vi "CRYO_MASTER_FULL_RUN3.vi"() -> ()   [LabVIEW 2017] (continued)
              }
              frame #1 {
                w484 = "_" ("string")
                n232 = local read "Cycle #"() -> (w482:u32)
                n233 = call "LV_UNIXTIME.vi"("current time"=w474) -> ("date/time string"=w485:string)  [unwired: 9 in, 1 out]
                n234 = Format Value(format string="%06d", value (0)=w482) -> (output string=w481:string)  [unwired: 1 in]
                n235 = Concatenate Strings(w472, w485, w484, w481, w484, "page5.png" ("string")) -> (w479:string)
                n236 = invoke class="TabCtl (strict)" method="Get Image"(error in=errorcluster {"status"=FALSE, "code"=0, "source"=""} ("error in (no error)")) -> (error out=w475:errorcluster, "image data"=w477:T23)  [unwired: 5 in, 4 out]
                n237 = Build Path(base path=w486, name or relative path=w479) -> (appended path=w478:path)
                n238 = call <vilib>:"Write PNG File.vi"("error in (no error)"=w475, "image data"=w477, "path to PNG file"=w478) -> ("error out"=w473:errorcluster)  [unwired: 7 in, 1 out]
              }
            }
            n239 = local write "error out (frontpanel screenshots)"(w466) -> ()
          }
          frame #5 {
            n240 = flat-sequence {
              tunnel: w490 -> [w493]
              tunnel: [w493] -> w489
              tunnel: w491 -> [w508]
              tunnel: w489 -> [w496]
              tunnel: [w495] -> w488
              tunnel: w487 -> [w494]
              frame #0 {
                n241 = property class="TabCtl (strict)"("Val(Sgnl)"=T1."DMMs" ("Value (Signaling)")) -> ()  [unwired: 2 in, 2 out]
              }
              frame #1 {
                w506 = "_" ("string")
                n242 = local read "Cycle #"() -> (w504:u32)
                n243 = call "LV_UNIXTIME.vi"("current time"=w496) -> ("date/time string"=w507:string)  [unwired: 9 in, 1 out]
                n244 = Format Value(format string="%06d", value (0)=w504) -> (output string=w503:string)  [unwired: 1 in]
                n245 = Concatenate Strings(w494, w507, w506, w503, w506, "page6.png" ("string")) -> (w501:string)
                n246 = invoke class="TabCtl (strict)" method="Get Image"(error in=errorcluster {"status"=FALSE, "code"=0, "source"=""} ("error in (no error)")) -> (error out=w497:errorcluster, "image data"=w499:T23)  [unwired: 5 in, 4 out]
                n247 = Build Path(base path=w508, name or relative path=w501) -> (appended path=w500:path)
                n248 = call <vilib>:"Write PNG File.vi"("error in (no error)"=w497, "image data"=w499, "path to PNG file"=w500) -> ("error out"=w495:errorcluster)  [unwired: 7 in, 1 out]
              }
            }
            n249 = local write "error out (frontpanel screenshots)"(w488) -> ()
          }
          frame #6 {
            n250 = flat-sequence {
              tunnel: w512 -> [w515]
              tunnel: [w515] -> w511
              tunnel: w513 -> [w530]
              tunnel: w511 -> [w518]
              tunnel: [w517] -> w510
              tunnel: w509 -> [w516]
              frame #0 {
                n251 = property class="TabCtl (strict)"("Val(Sgnl)"=T1."DIAGRAM" ("Value (Signaling)")) -> ()  [unwired: 2 in, 2 out]
              }
              frame #1 {
                w528 = "_" ("string")
                n252 = local read "Cycle #"() -> (w526:u32)
                n253 = Format Value(format string="%06d", value (0)=w526) -> (output string=w525:string)  [unwired: 1 in]
                n254 = call "LV_UNIXTIME.vi"("current time"=w518) -> ("date/time string"=w529:string)  [unwired: 9 in, 1 out]
                n255 = Concatenate Strings(w516, w529, w528, w525, w528, "page7.png" ("string")) -> (w523:string)
                n256 = invoke class="TabCtl (strict)" method="Get Image"(error in=errorcluster {"status"=FALSE, "code"=0, "source"=""} ("error in (no error)")) -> (error out=w519:errorcluster, "image data"=w521:T23)  [unwired: 5 in, 4 out]
                n257 = Build Path(base path=w530, name or relative path=w523) -> (appended path=w522:path)
                n258 = call <vilib>:"Write PNG File.vi"("error in (no error)"=w519, "image data"=w521, "path to PNG file"=w522) -> ("error out"=w517:errorcluster)  [unwired: 7 in, 1 out]
              }
            }
            n259 = local write "error out (frontpanel screenshots)"(w510) -> ()
          }
          frame #7 {
            n260 = flat-sequence {
              tunnel: w534 -> [w537]
              tunnel: [w537] -> w533
              tunnel: w535 -> [w552]
              tunnel: w533 -> [w540]
              tunnel: [w539] -> w532
              tunnel: w531 -> [w538]
              frame #0 {
                n261 = property class="TabCtl (strict)"("Val(Sgnl)"=T1."CHF" ("Value (Signaling)")) -> ()  [unwired: 2 in, 2 out]
              }
              frame #1 {
                w550 = "_" ("string")
                n262 = local read "Cycle #"() -> (w548:u32)
                n263 = Format Value(format string="%06d", value (0)=w548) -> (output string=w547:string)  [unwired: 1 in]
                n264 = call "LV_UNIXTIME.vi"("current time"=w540) -> ("date/time string"=w551:string)  [unwired: 9 in, 1 out]
                n265 = Concatenate Strings(w538, w551, w550, w547, w550, "page8.png" ("string")) -> (w545:string)
                n266 = invoke class="TabCtl (strict)" method="Get Image"(error in=errorcluster {"status"=FALSE, "code"=0, "source"=""} ("error in (no error)")) -> (error out=w541:errorcluster, "image data"=w543:T23)  [unwired: 5 in, 4 out]
                n267 = Build Path(base path=w552, name or relative path=w545) -> (appended path=w544:path)
                n268 = call <vilib>:"Write PNG File.vi"("error in (no error)"=w541, "image data"=w543, "path to PNG file"=w544) -> ("error out"=w539:errorcluster)  [unwired: 7 in, 1 out]
              }
            }
            n269 = local write "error out (frontpanel screenshots)"(w532) -> ()
          }
          frame #8 {
            n270 = flat-sequence {
              tunnel: w556 -> [w559]
              tunnel: [w559] -> w555
              tunnel: w557 -> [w574]
              tunnel: w555 -> [w562]
              tunnel: [w561] -> w554
              tunnel: w553 -> [w560]
              frame #0 {
                n271 = property class="TabCtl (strict)"("Val(Sgnl)"=T1."(Plc. hld.)" ("Value (Signaling)")) -> ()  [unwired: 2 in, 2 out]
              }
              frame #1 {
                w572 = "_" ("string")
                n272 = local read "Cycle #"() -> (w570:u32)
                n273 = Format Value(format string="%06d", value (0)=w570) -> (output string=w569:string)  [unwired: 1 in]
                n274 = call "LV_UNIXTIME.vi"("current time"=w562) -> ("date/time string"=w573:string)  [unwired: 9 in, 1 out]
                n275 = Concatenate Strings(w560, w573, w572, w569, w572, "page8.png" ("string")) -> (w567:string)
                n276 = invoke class="TabCtl (strict)" method="Get Image"(error in=errorcluster {"status"=FALSE, "code"=0, "source"=""} ("error in (no error)")) -> (error out=w563:errorcluster, "image data"=w565:T23)  [unwired: 5 in, 4 out]
                n277 = Build Path(base path=w574, name or relative path=w567) -> (appended path=w566:path)
                n278 = call <vilib>:"Write PNG File.vi"("error in (no error)"=w563, "image data"=w565, "path to PNG file"=w566) -> ("error out"=w561:errorcluster)  [unwired: 7 in, 1 out]
              }
            }
            n279 = local write "error out (frontpanel screenshots)"(w554) -> ()
          }
          frame #9 {
            n280 = local write "Frontpanel screenshots"(FALSE ("Frontpanel screenshots")) -> ()
          }
        }
        "error out (frontpanel screenshots)" <- w373
        n281 = property class="TabCtl (strict)"("Val(Sgnl)"=w371) -> ()  [unwired: 2 in, 2 out]
      }
      event "Stop Button": Value Change {
        n282 = event-data() -> ()  [unwired: 1 in, 3 out]
      }
    }
    n283 = Wait (ms)(milliseconds to wait=u32 123) -> ()  [unwired: 1 out]
  }
  n284 = while {
    stop <- w581 stop-if-true
    n285 = event shown="[5] \"Plot selecter LSI218(1)     1      2     3     4\", \"Plot selecter LSI218(2)     1      2     3     4\", \"Plot selecter (USB6210)     1      2     3     4\", \"Plot selecter LSI336       1      2     3     4\", \"Plot selecter (USB6218)     1      2     3     4\", \"Plot selecter (HP34401A)     1      2     3     4\": Value Change" {
      selector: _ -> [_ _ _ _ _ _ _ _ _ _ _]
      dyn-events: _ -> [_ _ _ _ _ _ _ _ _ _ _]
      timeout: _ -> [_ _ _ _ _ _ _ _ _ _ _]
      tunnel: [_ _ _ _ _ _ _ _ _ _ TRUE] -> w581
      tunnel: [errorcluster {"status"=FALSE, "code"=0, "source"=""} ("error out") w585 _ _ _ _ w721 w738 w755 w772 errorcluster {"status"=FALSE, "code"=0, "source"=""} ("error out")] -> w577
      event Timeout {
        n286 = event-data() -> ()  [unwired: 1 in, 3 out]
      }
      event "log/linear 1": Value Change {
        n287 = event-data() -> ()  [unwired: 1 in, 6 out]
        n288 = flat-sequence {
          tunnel: [w586] -> w585
          frame #0 {
            n289 = Boolean To (0,1)(Boolean="log/linear 1") -> (0, 1=w591:i16)
            n290 = control-ref of="Graph 1"() -> (w587:refnum<vi>)
            n291 = property class="XYGraph (strict)"(reference=w587, error in=errorcluster {"status"=FALSE, "code"=0, "source"=""} ("error in (no error)"), "YScale.Mapping Mode"=w591) -> (error out=w589:errorcluster)  [unwired: 1 out]
            n292 = control-ref of="error out (USB6210)"() -> (w590:refnum<vi>)
            n293 = property class="Clust (strict)"(reference=w590, "Val(Sgnl)"=w589) -> (error out=w586:errorcluster)  [unwired: 1 in, 1 out]
          }
        }
      }
      event "log/linear 2": Value Change {
        n294 = event-data() -> ()  [unwired: 1 in, 6 out]
        n295 = flat-sequence {
          frame #0 {
            n296 = Boolean To (0,1)(Boolean="log/linear 2") -> (0, 1=w597:i16)
            n297 = control-ref of="Graph 2"() -> (w595:refnum<vi>)
            n298 = property class="XYGraph (strict)"(reference=w595, error in=errorcluster {"status"=FALSE, "code"=0, "source"=""} ("error in (no error)"), "YScale.Mapping Mode"=w597) -> (error out=w596:errorcluster)  [unwired: 1 out]
            n299 = control-ref of="error out (USB6210)"() -> (w594:refnum<vi>)
            n300 = property class="Clust (strict)"(reference=w594, "Value"=w596) -> ()  [unwired: 1 in, 2 out]
          }
        }
      }
      event "log/linear 3": Value Change {
        n301 = event-data() -> ()  [unwired: 1 in, 6 out]
        n302 = flat-sequence {
          frame #0 {
            n303 = Boolean To (0,1)(Boolean="log/linear 3") -> (0, 1=w603:i16)
            n304 = control-ref of="Graph 3"() -> (w599:refnum<vi>)
            n305 = property class="XYGraph (strict)"(reference=w599, error in=errorcluster {"status"=FALSE, "code"=0, "source"=""} ("error in (no error)"), "YScale.Mapping Mode"=w603) -> (error out=w602:errorcluster)  [unwired: 1 out]
            n306 = control-ref of="error out (USB6210)"() -> (w601:refnum<vi>)
            n307 = property class="Clust (strict)"(reference=w601, "Value"=w602) -> ()  [unwired: 1 in, 2 out]
          }
        }
      }
      event "log/linear 4": Value Change {
        n308 = event-data() -> ()  [unwired: 1 in, 6 out]
        n309 = flat-sequence {
          frame #0 {
            n310 = Boolean To (0,1)(Boolean="log/linear 4") -> (0, 1=w609:i16)
            n311 = control-ref of="Graph 4"() -> (w605:refnum<vi>)
            n312 = property class="XYGraph (strict)"(reference=w605, error in=errorcluster {"status"=FALSE, "code"=0, "source"=""} ("error in (no error)"), "YScale.Mapping Mode"=w609) -> (error out=w608:errorcluster)  [unwired: 1 out]
            n313 = control-ref of="error out (USB6210)"() -> (w607:refnum<vi>)
            n314 = property class="Clust (strict)"(reference=w607, "Value"=w608) -> ()  [unwired: 1 in, 2 out]
          }
        }
      }
      event "Plot selecter LSI218(1)\n    1      2     3     4", "Plot selecter LSI218(2)\n    1      2     3     4", "Plot selecter (USB6210)\n    1      2     3     4", "Plot selecter LSI336 \n     1      2     3     4", "Plot selecter (USB6218)\n    1      2     3     4", "Plot selecter (HP34401A)\n    1      2     3     4": Value Change {
        n315 = event-data() -> ()  [unwired: 1 in, 6 out]
        n316 = local read "Labels (HP34401 LM)"() -> (w616:string[])
        n317 = call "BuildPlotLegends.vi"("Plot selecter \n    1      2     3     4"="Plot selecter (HP34401A)\n    1      2     3     4", "AllLabels"=w616) -> ("Series 4"=w611:string[], "Series 3"=w612:string[], "Series 2"=w613:string[], "Series 1"=w614:string[])  [unwired: 6 in]
        n318 = local read "All Labels (USB6210)"() -> (w633:string[])
        n319 = local read "All Labels (USB6218)"() -> (w622:string[])
        n320 = local read "Labels LSI218 (1)"() -> (w635:string[])
        n321 = local read "Labels LSI218 (2)"() -> (w636:string[])
        n322 = local read "Labels LSI336"() -> (w628:string[])
        n323 = call "BuildPlotLegends_LSI218.vi"("Plot selecter (2)\n    1      2     3     5"="Plot selecter LSI218(2)\n    1      2     3     4", "Plot selecter (1)\n    1      2     3     4"="Plot selecter LSI218(1)\n    1      2     3     4", "Labels (2)"=w636, "Labels (1)"=w635) -> ("Series 4"=w646:string[], "Series 3"=w644:string[], "Series 2"=w642:string[], "Series 1"=w640:string[])  [unwired: 4 in]
        n324 = call "BuildPlotLegends.vi"("Plot selecter \n    1      2     3     4"="Plot selecter (USB6210)\n    1      2     3     4", "AllLabels"=w633) -> ("Series 4"=w645:string[], "Series 3"=w643:string[], "Series 2"=w641:string[], "Series 1"=w639:string[])  [unwired: 6 in]
        n325 = call "BuildPlotLegends.vi"("Plot selecter \n    1      2     3     4"="Plot selecter LSI336 \n     1      2     3     4", "AllLabels"=w628) -> ("Series 4"=w623:string[], "Series 3"=w624:string[], "Series 2"=w625:string[], "Series 1"=w626:string[])  [unwired: 6 in]
        n326 = call "BuildPlotLegends.vi"("Plot selecter \n    1      2     3     4"="Plot selecter (USB6218)\n    1      2     3     4", "AllLabels"=w622) -> ("Series 4"=w618:string[], "Series 3"=w617:string[], "Series 2"=w619:string[], "Series 1"=w620:string[])  [unwired: 6 in]
        n327 = Build Array (concatenate)(w641, w642, w625, w619, w613) -> (w630:string[])
        "Series 2" <- w630
        n328 = Build Array (concatenate)(w643, w644, w624, w617, w612) -> (w631:string[])
        "Series 3" <- w631
        n329 = Build Array (concatenate)(w645, w646, w623, w618, w611) -> (w632:string[])
        "Series 4" <- w632
        n330 = Build Array (concatenate)(w639, w640, w626, w620, w614) -> (w629:string[])
        "Series 1" <- w629
        n331 = stacked-sequence {
          tunnel: [w656 _ _ _] -> w650
          tunnel: [_ w674 _ _] -> w651
          tunnel: [_ _ w691 _] -> w649
          tunnel: [_ _ _ w708] -> w648
          tunnel: w629 -> [w654 _ _ _]
          tunnel: w630 -> [_ w672 _ _]
          tunnel: w631 -> [_ _ w689 _]
          tunnel: w632 -> [_ _ _ w706]
          frame #0 {
            n332 = Array Size(array=w654) -> (size(s)=w658:i32)
            n333 = control-ref of="Graph 1"() -> (w652:refnum<vi>)
            n334 = property class="XYGraph (strict)"(reference=w652) -> ("LegNumRows"=w653:u32)  [unwired: 1 in, 2 out]
            n335 = for {
              N: w653 -> [_]
              tunnel: w652 -> [w667]
              shift-right: [w665] -> w657
              shift-left: errorcluster {"status"=FALSE, "code"=0, "source"=""} ("error in (no error)") -> [w666]
              i -> [w669]
              n336 = property class="XYGraph (strict)"(reference=w667, error in=w666, "Active Plot"=w669, "Plot.Plot Name"="") -> (error out=w665:errorcluster)  [unwired: 1 out]
            }
            n337 = for {
              N: w658 -> [_]
              tunnel: w652 -> [w663]
              shift-right: [w661] -> w656
              shift-left: w657 -> [w662]
              tunnel: w654 -> [w660] mode=indexing
              i -> [w664]
              n338 = property class="XYGraph (strict)"(reference=w663, error in=w662, "Active Plot"=w664, "Plot.Plot Name"=w660, "Plot.Visible?"=TRUE ("Plot.Visible")) -> (error out=w661:errorcluster)  [unwired: 1 out]
            }
          }
          frame #1 {
            n339 = Array Size(array=w672) -> (size(s)=w676:i32)
            n340 = control-ref of="Graph 2"() -> (w671:refnum<vi>)
            n341 = property class="XYGraph (strict)"(reference=w671) -> ("LegNumRows"=w670:u32)  [unwired: 1 in, 2 out]
            n342 = for {
              N: w670 -> [_]
              shift-right: [w683] -> w675
              shift-left: errorcluster {"status"=FALSE, "code"=0, "source"=""} ("error in (no error)") -> [w684]
              tunnel: w671 -> [w682]
              i -> [w686]
              n343 = property class="XYGraph (strict)"(reference=w682, error in=w684, "Active Plot"=w686, "Plot.Plot Name"="") -> (error out=w683:errorcluster)  [unwired: 1 out]
            }
            n344 = for {
              N: w676 -> [_]
              shift-right: [w679] -> w674
              shift-left: w675 -> [w680]
              tunnel: w672 -> [w678] mode=indexing
              tunnel: w671 -> [w677]
              i -> [w681]
              n345 = property class="XYGraph (strict)"(reference=w677, error in=w680, "Active Plot"=w681, "Plot.Plot Name"=w678) -> (error out=w679:errorcluster)  [unwired: 1 out]
            }
          }
          frame #2 {
            n346 = Array Size(array=w689) -> (size(s)=w693:i32)
            n347 = control-ref of="Graph 3"() -> (w687:refnum<vi>)
            n348 = property class="XYGraph (strict)"(reference=w687) -> ("LegNumRows"=w688:u32)  [unwired: 1 in, 2 out]
            n349 = for {
              N: w688 -> [_]
              tunnel: w687 -> [w701]
              shift-right: [w699] -> w692
              shift-left: errorcluster {"status"=FALSE, "code"=0, "source"=""} ("error in (no error)") -> [w700]
              i -> [w703]
              n350 = property class="XYGraph (strict)"(reference=w701, error in=w700, "Active Plot"=w703, "Plot.Plot Name"="") -> (error out=w699:errorcluster)  [unwired: 1 out]
            }
            n351 = for {
              N: w693 -> [_]
              tunnel: w687 -> [w697]
              shift-right: [w695] -> w691
              shift-left: w692 -> [w696]
              tunnel: w689 -> [w694] mode=indexing
              i -> [w698]
              n352 = property class="XYGraph (strict)"(reference=w697, error in=w696, "Active Plot"=w698, "Plot.Plot Name"=w694) -> (error out=w695:errorcluster)  [unwired: 1 out]
            }
          }
          frame #3 {
            n353 = Array Size(array=w706) -> (size(s)=w710:i32)
            n354 = control-ref of="Graph 4"() -> (w704:refnum<vi>)
            n355 = property class="XYGraph (strict)"(reference=w704) -> ("LegNumRows"=w705:u32)  [unwired: 1 in, 2 out]
            n356 = for {
              N: w705 -> [_]
              tunnel: w704 -> [w718]
              shift-right: [w716] -> w709
              shift-left: errorcluster {"status"=FALSE, "code"=0, "source"=""} ("error in (no error)") -> [w717]
              i -> [w720]
              n357 = property class="XYGraph (strict)"(reference=w718, error in=w717, "Active Plot"=w720, "Plot.Plot Name"="") -> (error out=w716:errorcluster)  [unwired: 1 out]
            }
            n358 = for {
              N: w710 -> [_]
              tunnel: w704 -> [w714]
              shift-right: [w712] -> w708
              shift-left: w709 -> [w713]
              tunnel: w706 -> [w711] mode=indexing
              i -> [w715]
              n359 = property class="XYGraph (strict)"(reference=w714, error in=w713, "Active Plot"=w715, "Plot.Plot Name"=w711) -> (error out=w712:errorcluster)  [unwired: 1 out]
            }
          }
        }
        n360 = Merge Errors(w650, w651, w649, w648) -> (→"Plot errors":errorcluster)
      }
      event "Take Screenshot! 1": Value Change {
        n361 = event-data() -> ()  [unwired: 1 in, 6 out]
        n362 = flat-sequence {
          tunnel: [w722] -> w721
          frame #0 {
            n363 = flat-sequence {
              tunnel: [w723] -> w722
              frame #0 {
                w732 = "_" ("string")
                n364 = Get Date/Time In Seconds() -> (seconds since 1Jan1904=w729:timestamp)
                n365 = local read "RUN Identifier"() -> (w734:string)
                n366 = call "LV_UNIXTIME.vi"("current time"=w729) -> ("date/time string"=w733:string)  [unwired: 9 in, 1 out]
                n367 = control-ref of="Graph 1"() -> (w728:refnum<vi>)
                n368 = Concatenate Strings(w734, w732, w733, w732, "FIle suffix 1", ".png" ("string")) -> (w736:string)
                n369 = local read "Base Path"() -> (w735:path)
                n370 = invoke class="XYGraph (strict)" method="Get Image"(reference=w728, error in=errorcluster {"status"=FALSE, "code"=0, "source"=""} ("error in (no error)")) -> (error out=w724:errorcluster, "image data"=w727:T23)  [unwired: 4 in, 4 out]
                n371 = Build Path(base path=w735, name or relative path=w736) -> (appended path=w726:path)
                n372 = call <vilib>:"Write PNG File.vi"("error in (no error)"=w724, "image data"=w727, "path to PNG file"=w726) -> ("error out"=w723:errorcluster)  [unwired: 7 in, 1 out]
              }
              frame #1 {
                n373 = local write "Take Screenshot! 1"(FALSE ("Take Screenshot! 1")) -> ()
              }
            }
          }
        }
      }
      event "Take Screenshot! 2": Value Change {
        n374 = event-data() -> ()  [unwired: 1 in, 6 out]
        n375 = flat-sequence {
          tunnel: [w739] -> w738
          frame #0 {
            n376 = flat-sequence {
              tunnel: [w745] -> w739
              frame #0 {
                w749 = "_" ("string")
                n377 = Get Date/Time In Seconds() -> (seconds since 1Jan1904=w746:timestamp)
                n378 = local read "RUN Identifier"() -> (w751:string)
                n379 = call "LV_UNIXTIME.vi"("current time"=w746) -> ("date/time string"=w750:string)  [unwired: 9 in, 1 out]
                n380 = control-ref of="Graph 2"() -> (w740:refnum<vi>)
                n381 = Concatenate Strings(w751, w749, w750, w749, "FIle suffix 2", ".png" ("string")) -> (w753:string)
                n382 = local read "Base Path"() -> (w752:path)
                n383 = invoke class="XYGraph (strict)" method="Get Image"(reference=w740, error in=errorcluster {"status"=FALSE, "code"=0, "source"=""} ("error in (no error)")) -> (error out=w744:errorcluster, "image data"=w742:T23)  [unwired: 4 in, 4 out]
                n384 = Build Path(base path=w752, name or relative path=w753) -> (appended path=w741:path)
                n385 = call <vilib>:"Write PNG File.vi"("error in (no error)"=w744, "image data"=w742, "path to PNG file"=w741) -> ("error out"=w745:errorcluster)  [unwired: 7 in, 1 out]
              }
              frame #1 {
                n386 = local write "Take Screenshot! 2"(FALSE ("Take Screenshot! 1")) -> ()
              }
            }
          }
        }
      }
      event "Take Screenshot! 3": Value Change {
        n387 = event-data() -> ()  [unwired: 1 in, 6 out]
        n388 = flat-sequence {
          tunnel: [w756] -> w755
          frame #0 {
            n389 = flat-sequence {
              tunnel: [w758] -> w756
              frame #0 {
                w766 = "_" ("string")
                n390 = Get Date/Time In Seconds() -> (seconds since 1Jan1904=w764:timestamp)
                n391 = local read "RUN Identifier"() -> (w768:string)
                n392 = call "LV_UNIXTIME.vi"("current time"=w764) -> ("date/time string"=w767:string)  [unwired: 9 in, 1 out]
                n393 = control-ref of="Graph 3"() -> (w761:refnum<vi>)
                n394 = Concatenate Strings(w768, w766, w767, w766, "FIle suffix 3", ".png" ("string")) -> (w770:string)
                n395 = local read "Base Path"() -> (w769:path)
                n396 = invoke class="XYGraph (strict)" method="Get Image"(reference=w761, error in=errorcluster {"status"=FALSE, "code"=0, "source"=""} ("error in (no error)")) -> (error out=w759:errorcluster, "image data"=w757:T23)  [unwired: 4 in, 4 out]
                n397 = Build Path(base path=w769, name or relative path=w770) -> (appended path=w762:path)
                n398 = call <vilib>:"Write PNG File.vi"("error in (no error)"=w759, "image data"=w757, "path to PNG file"=w762) -> ("error out"=w758:errorcluster)  [unwired: 7 in, 1 out]
              }
              frame #1 {
                n399 = local write "Take Screenshot! 3"(FALSE ("Take Screenshot! 1")) -> ()
              }
            }
          }
        }
      }
      event "Take Screenshot! 4": Value Change {
        n400 = event-data() -> ()  [unwired: 1 in, 6 out]
        n401 = flat-sequence {
          tunnel: [w773] -> w772
          frame #0 {
            n402 = flat-sequence {
              tunnel: [w776] -> w773
              frame #0 {
                w783 = "_" ("string")
                n403 = Get Date/Time In Seconds() -> (seconds since 1Jan1904=w781:timestamp)
                n404 = local read "RUN Identifier"() -> (w785:string)
                n405 = call "LV_UNIXTIME.vi"("current time"=w781) -> ("date/time string"=w784:string)  [unwired: 9 in, 1 out]
                n406 = control-ref of="Graph 4"() -> (w777:refnum<vi>)
                n407 = Concatenate Strings(w785, w783, w784, w783, "FIle suffix 4", ".png" ("string")) -> (w787:string)
                n408 = local read "Base Path"() -> (w786:path)
                n409 = invoke class="XYGraph (strict)" method="Get Image"(reference=w777, error in=errorcluster {"status"=FALSE, "code"=0, "source"=""} ("error in (no error)")) -> (error out=w774:errorcluster, "image data"=w778:T23)  [unwired: 4 in, 4 out]
                n410 = Build Path(base path=w786, name or relative path=w787) -> (appended path=w779:path)
                n411 = call <vilib>:"Write PNG File.vi"("error in (no error)"=w774, "image data"=w778, "path to PNG file"=w779) -> ("error out"=w776:errorcluster)  [unwired: 7 in, 1 out]
              }
              frame #1 {
                n412 = local write "Take Screenshot! 4"(FALSE ("Take Screenshot! 1")) -> ()
              }
            }
          }
        }
      }
      event "Stop Button": Value Change {
        n413 = event-data() -> ()  [unwired: 1 in, 6 out]
      }
    }
    "error out (graph operations)" <- w577
    n414 = local write "Take Screenshot! 1"(FALSE ("Take Screenshot! 1")) -> ()
    n415 = local write "Take Screenshot! 2"(FALSE ("Take Screenshot! 1")) -> ()
    n416 = Wait (ms)(milliseconds to wait=u32 1000) -> ()  [unwired: 1 out]
    n417 = local write "Take Screenshot! 3"(FALSE ("Take Screenshot! 1")) -> ()
    n418 = local write "Take Screenshot! 4"(FALSE ("Take Screenshot! 1")) -> ()
  }
  n419 = while {
    i -> [w795]
    stop <- w792 stop-if-true
    n420 = Equal?(x=w795, y=0) -> (x = y?=w793:bool)
    n421 = case shown="True" w793 {
      frame False {
      }
      frame True {
        n422 = property on="Agilent\nIntialized?" class="Bool (strict)"("Val(Sgnl)"=FALSE ("Value (Signaling)")) -> ()  [unwired: 2 in, 2 out]
      }
    }
    n423 = Wait (ms)(milliseconds to wait=u32 123) -> ()  [unwired: 1 out]
    n424 = event shown="[4] \"V_lim_up (V)\", \"V_lim_low (V)\": Value Change" {
      selector: _ -> [_ _ _ _ _]
      dyn-events: _ -> [_ _ _ _ _]
      timeout: _ -> [_ _ _ _ _]
      tunnel: [FALSE ("Value (Signaling)") TRUE ("Value (Signaling)") _ _ _] -> w792
      tunnel: "VISA (Agilent 34402)" -> [_ _ w801 w804 _]
      event Timeout {
        n425 = event-data() -> ()  [unwired: 1 in, 3 out]
      }
      event "Stop Button": Value Change {
        n426 = event-data() -> ()  [unwired: 1 in, 3 out]
      }
      event "Initialize (Agilent)": Value Change {
        n427 = event-data() -> ()  [unwired: 1 in, 3 out]
        n428 = property on="Agilent\nIntialized?" class="Bool (strict)"("Val(Sgnl)"=TRUE ("Value (Signaling)")) -> ()  [unwired: 2 in, 2 out]
        n429 = call "Initialize.vi"("error in (no error)"=errorcluster {"status"=FALSE, "code"=0, "source"=""}, "VISA resource name"=w801) -> ("error out"=→"error out (Agilent)":errorcluster)  [unwired: 8 in, 1 out]
      }
      event "OUTPUT \nKenwood", "Kenwood set V (V)": Value Change {
        n430 = local read "Agilent\nIntialized?"() -> (w803:bool)
        n431 = event-data() -> ()  [unwired: 1 in, 3 out]
        n432 = case shown="True" w803 {
          tunnel: w804 -> [_ w810]
          frame False {
          }
          frame True {
            w812 = u16 0 items=["DC", "Sine", "Square", "Triangle", "Ramp", "Pulse", "Noise", "Sinc", "Negative Ramp", "Exponential Rise", "Exponential Fall", "Cardiac"] ("Waveform Function (1: Sine)")
            n433 = xnode "Formula"("X1"="Kenwood set V (V)") -> ("Result"=w805:dbl)  [unwired: 1 in, 1 out]
            n434 = call "Configure Standard Waveform.vi"("DC Offset (0.00 V)"=w805, "Frequency (1000 Hz)"=1.0, "error in (no error)"=errorcluster {"status"=FALSE, "code"=0, "source"=""}, "Amplitude (1)"=1.0, "Waveform Function (1: Sine)"=w812, "VISA resource name"=w810) -> ("error out"=w814:errorcluster, "VISA resource name out"=w815:refnum<visa-resource-name>)  [unwired: 4 in]
            n435 = call "Enable Output.vi"("error in (no error)"=w814, "Enable Output  (T: Enable)"="OUTPUT \nKenwood", "VISA resource name"=w815) -> ("error out"=w808:errorcluster)  [unwired: 7 in, 1 out]
            n436 = local write "error out (Agilent)"(w808) -> ()
          }
        }
      }
      event "V_lim_up (V)", "V_lim_low (V)": Value Change {
        n437 = event-data() -> ()  [unwired: 1 in, 3 out]
        n438 = property on="Kenwood set V (V)" class="DigNum (strict)"("Minimum"="V_lim_low (V)", "Maximum"="V_lim_up (V)") -> ()  [unwired: 2 in, 2 out]
      }
    }
  }
  n439 = while {
    stop <- w827 stop-if-true
    n440 = Wait (ms)(milliseconds to wait=u32 101) -> ()  [unwired: 1 out]
    n441 = event shown="[2] Timeout" {
      selector: _ -> [_ _ _]
      dyn-events: _ -> [_ _ _]
      timeout: _ -> [_ _ _]
      tunnel: [FALSE TRUE FALSE] -> w827
      event "Initialize (DMMs)": Value Change {
        w830 = T4 [] ("Value (Signaling)")
        n442 = event-data() -> ()  [unwired: 1 in, 3 out]
        n443 = property on="Graph DMMs 1" class="XYGraph (strict)"("Val(Sgnl)"=w830) -> ()  [unwired: 2 in, 2 out]
        n444 = property on="Graph DMMs 2" class="XYGraph (strict)"("Val(Sgnl)"=w830) -> ()  [unwired: 2 in, 2 out]
      }
      event "Stop Button": Value Change {
        n445 = event-data() -> ()  [unwired: 1 in, 3 out]
      }
      event Timeout {
        n446 = event-data() -> ()  [unwired: 1 in, 3 out]
      }
    }
  }
  n447 = Obtain Notifier(name (unnamed)="stop notifier", notification data type=w17, create if not found? (T)=w17, error in (no error)=errorcluster {"status"=FALSE, "code"=0, "source"=""}) -> (notifier out=w5:refnum<notifier>, error out=w4:errorcluster)  [unwired: 1 out]
  n448 = while {
    shift-right: [w943] -> w40
    shift-left: refnum<class "USBData.lvclass"> refnum ("USBData.lvclass") -> [w946]
    shift-right: [w939] -> w39
    shift-left: w6 -> [w945]
    tunnel: "Base Path" -> [w845]
    shift-right: [w921] -> w34
    shift-left: errorcluster {"status"=FALSE, "code"=0, "source"=""} ("error in (no error)") -> [w937]
    shift-right: [w922] -> w35
    shift-left: refnum<class "LSI218Data.lvclass"> refnum ("LSI218Data.lvclass") -> [w936]
    shift-right: [w909] -> w31
    shift-left: refnum<class "LSI336Data.lvclass"> refnum ("LSI336Data.lvclass") -> [w918]
    shift-right: [w908] -> w30
    shift-left: w21 -> [w917]
    shift-right: [w897] -> _
    shift-left: w6 -> [w898]
    shift-right: [w887] -> w25
    shift-left: refnum<class "USBData.lvclass"> refnum ("USBData.lvclass") -> [w895]
    shift-right: [w886] -> w24
    shift-left: errorcluster {"status"=FALSE, "code"=0, "source"=""} ("error in (no error)") -> [w894]
    shift-right: [w883] -> _
    shift-left: w21 -> [w882]
    tunnel: w5 -> [w853]
    tunnel: w4 -> [w852]
    tunnel: [w850] -> w13
    tunnel: [w849] -> w12
    shift-right: [w846] -> _
    shift-left: refnum<class "LMData.lvclass"> refnum ("LMData in") -> [w847]
    shift-right: [w843] -> _
    shift-left: errorcluster {"status"=FALSE, "code"=0, "source"=""} ("error in (no error)") -> [w844]
    i -> [w842]
    stop <- "Stop Button" stop-if-true
    w838 = T25 [] ("appended array")
    w904 = u32 24 ("Number of Rows")
    w914 = T25 [] ("appended array")
    w931 = T25 [] ("appended array")
    n449 = local read "LSI218Settings(A-F)"() -> (w874:T3)
    n450 = control-ref of="Plot selecter LSI218(2)\n    1      2     3     4"() -> (w902:refnum<vi>)
    n451 = control-ref of="Plot selecter LSI218(1)\n    1      2     3     4"() -> (w903:refnum<vi>)
    n452 = control-ref of="Plot selecter LSI336 \n     1      2     3     4"() -> (w901:refnum<vi>)
    n453 = property on="Property Node" class="Arr (strict)"(reference=w902, "Number of Rows"=w904) -> ()  [unwired: 1 in, 2 out]
    n454 = property on="Property Node" class="Arr (strict)"(reference=w903, "Number of Rows"=w904) -> ()  [unwired: 1 in, 2 out]
    n455 = local read "LSI336Settings(X,Y)"() -> (w872:T3)
    n456 = Array Size(array=w874) -> (size(s)=w873:i32)
    n457 = property on="Property Node" class="Arr (strict)"(reference=w901, "Number of Rows"=u32 8) -> ()  [unwired: 1 in, 2 out]
    n458 = Multiply(x="Measurement Interval (s)", y=u32 1000) -> (x*y=w940:dbl)
    n459 = Wait (ms)(milliseconds to wait=w940) -> ()  [unwired: 1 out]
    n460 = for {
      N: w873 -> [_]
      tunnel: w874 -> [w1034] mode=indexing
      tunnel: [w1033] -> w870 mode=concatenating
      n461 = Unbundle By Name(w1034) -> ("SensorLocations"=w1033:T18)
    }
    n462 = for {
      tunnel: w872 -> [w1032] mode=indexing
      tunnel: [w1031] -> w871 mode=concatenating
      n463 = Unbundle By Name(w1032) -> ("SensorLocations"=w1031:T18)
    }
    n464 = Quotient & Remainder(x=w842, y="Screenshots interval") -> (x-y*floor(x/y)=w858:i64)  [unwired: 1 out]
    n465 = Equal?(x=w842, y=0) -> (x = y?=w848:bool)
    n466 = case shown="True" w848 {
      tunnel: w946 -> [w2099 w2122]
      tunnel: w945 -> [w2093 w2120]
      tunnel: w842 -> [w2084 _]
      tunnel: [w2091 w2117] -> w939
      tunnel: [w2088 w2116] -> w896
      tunnel: [w2089 w2115] -> w943
      tunnel: [w2079 w2110] -> w944
      tunnel: w845 -> [_ w2109]
      tunnel: [w2078 w2106] -> w879
      frame False {
        n467 = call-dynamic "USBData_measure.vi"("USBData in"=w2099, "DAQ sample #"=i64 5, "DAQ timeout"=100.0 ("DAQ timeout (def: 100)"), "MeasurementIndex"=w2084, "error in (no error)"=w2093, "save every ... measurements"="Record interval") -> ("USBData out"=w2098:refnum<class "USBData.lvclass">, "TimeMeasuremeent"=w2095:timestamp, "Status"=→"USB6210 Status":T6, "LastDataAcquired"=w2080:dbl[], "error out"=w2094:errorcluster)  [unwired: 3 in, 2 out]
        "Time of Last Measurement (USB6210)" <- w2095
        "Last Vol\n(USB6210)" <- w2080
        n468 = call-dynamic "USBData_convert.vi"("Save every ... measurements"="Record interval", "MeasurementIndex"=w2084, "error in (no error)"=w2094, "LastDataAcquired"=w2080, "TimeMeasuremeent"=w2095, "USBData in"=w2098) -> ("error out"=w2092:errorcluster, "LeakDet_FULL"=w2087:dbl, "LastDataConverted"=w2081:dbl[], "USBData out"=w2090:refnum<class "USBData.lvclass">)  [unwired: 2 in]
        n469 = call "USBData_read.vi"("USBData in"=w2090, "error in (no error)"=w2092) -> ("Status"=w2082:T6, "USBData out"=w2089:refnum<class "USBData.lvclass">, "Data"=w2088:T26, "Basic"=w2079:T27, "error out"=w2091:errorcluster)  [unwired: 2 in, 2 out]
        n470 = local write "USB6210 Status"(w2082) -> ()
        n471 = Unbundle By Name(w2079) -> ("ReadLeakDet?"=w2086:bool)
        n472 = Unbundle By Name(w2079) -> ("Labels"=w2078:string[])
        n473 = case shown="False" w2086 {
          tunnel: w2081 -> [w2100 w2103]
          tunnel: w2087 -> [_ w2102]
          tunnel: [w2100 w2101] -> w2085
          frame False {
          }
          frame True {
            n474 = Build Array (concatenate)(w2103, w2102) -> (w2101:dbl[])
          }
        }
        "Last Data \n(USB6210)" <- w2085
      }
      frame True {
        n475 = local read "RUN Identifier"() -> (w2104:string)
        n476 = call-dynamic "USBData_initialize.vi"("USBData in"=w2122, "SeriesSetting"="USB6210 Config", "BasePath"=w2109, "RunIdentifier"=w2104, "FileName"="InstName (USB6210)", "error in (no error)"=w2120) -> ("Status"=w2105:T6, "USBData out"=w2118:refnum<class "USBData.lvclass">, "error out"=w2119:errorcluster)  [unwired: 5 in, 2 out]
        n477 = local write "USB6210 Status"(w2105) -> ()
        n478 = call "USBData_read.vi"("USBData in"=w2118, "error in (no error)"=w2119) -> ("Status"=w2108:T6, "USBData out"=w2115:refnum<class "USBData.lvclass">, "Data"=w2116:T26, "Basic"=w2110:T27, "error out"=w2117:errorcluster)  [unwired: 2 in, 2 out]
        n479 = local write "USB6210 Status"(w2108) -> ()
        n480 = Unbundle By Name(w2110) -> ("ReadLeakDet?"=w2114:bool, "Labels"=w2106:string[])
        n481 = Array Size(array=w2106) -> (size(s)=w2113:i32)
        n482 = case shown="True" w2114 {
          tunnel: w2113 -> [w2123 w2125]
          tunnel: [w2123 w2124] -> w2111
          frame False {
          }
          frame True {
            n483 = Add(x=w2125, y=1) -> (x+y=w2124:i32)
          }
        }
        n484 = Initialize Array(TRUE ("Activate 2"), w2111) -> ()  [unwired: 1 out]
      }
    }
    "error out (USB6210)" <- w939
    n485 = case shown="False" w848 {
      tunnel: [w1615 w1642] -> w886
      tunnel: [w1612 w1641] -> w893
      tunnel: [w1613 w1640] -> w887
      tunnel: [w1604 w1635] -> w892
      tunnel: [w1603 w1633] -> _
      tunnel: w895 -> [w1602 w1631]
      tunnel: w845 -> [_ w1630]
      tunnel: w894 -> [w1601 w1629]
      tunnel: w842 -> [w1600 _]
      frame False {
        n486 = local read "Record interval"() -> (w1599:i64)
        n487 = call-dynamic "USBData_measure.vi"("USBData in"=w1602, "DAQ sample #"=i64 5, "DAQ timeout"=100.0 ("DAQ timeout (def: 100)"), "MeasurementIndex"=w1600, "error in (no error)"=w1601, "save every ... measurements"=w1599) -> ("USBData out"=w1621:refnum<class "USBData.lvclass">, "TimeMeasuremeent"=w1618:timestamp, "Status"=→"USB6218 Status":T6, "LastDataAcquired"=w1605:dbl[], "error out"=w1617:errorcluster)  [unwired: 3 in, 2 out]
        "Time of Last Measurement (USB6218)" <- w1618
        "Last Vol \n(USB6218)" <- w1605
        n488 = call-dynamic "USBData_convert.vi"("Save every ... measurements"=w1599, "MeasurementIndex"=w1600, "error in (no error)"=w1617, "LastDataAcquired"=w1605, "TimeMeasuremeent"=w1618, "USBData in"=w1621) -> ("error out"=w1616:errorcluster, "LeakDet_FULL"=w1611:dbl, "LastDataConverted"=w1606:dbl[], "USBData out"=w1614:refnum<class "USBData.lvclass">)  [unwired: 2 in]
        n489 = call "USBData_read.vi"("USBData in"=w1614, "error in (no error)"=w1616) -> ("Status"=w1607:T6, "USBData out"=w1613:refnum<class "USBData.lvclass">, "Data"=w1612:T26, "Basic"=w1604:T27, "error out"=w1615:errorcluster)  [unwired: 2 in, 2 out]
        n490 = local write "USB6218 Status"(w1607) -> ()
        n491 = Unbundle By Name(w1604) -> ("ReadLeakDet?"=w1610:bool)
        n492 = Unbundle By Name(w1604) -> ("Labels"=w1603:string[])
        n493 = case shown="True" w1610 {
          tunnel: w1606 -> [w1622 w1625]
          tunnel: w1611 -> [_ w1624]
          tunnel: [w1622 w1623] -> w1609
          frame False {
          }
          frame True {
            n494 = Build Array (concatenate)(w1625, w1624) -> (w1623:dbl[])
          }
        }
        "Last Data \n(USB6218)" <- w1609
      }
      frame True {
        n495 = local read "RUN Identifier"() -> (w1626:string)
        n496 = call-dynamic "USBData_initialize.vi"("USBData in"=w1631, "SeriesSetting"="USB6218 Config", "BasePath"=w1630, "RunIdentifier"=w1626, "FileName"="InstName (USB6218)", "error in (no error)"=w1629) -> ("Status"=w1627:T6, "USBData out"=w1643:refnum<class "USBData.lvclass">, "error out"=w1644:errorcluster)  [unwired: 5 in, 2 out]
        n497 = local write "USB6218 Status"(w1627) -> ()
        n498 = call "USBData_read.vi"("USBData in"=w1643, "error in (no error)"=w1644) -> ("Status"=w1634:T6, "USBData out"=w1640:refnum<class "USBData.lvclass">, "Data"=w1641:T26, "Basic"=w1635:T27, "error out"=w1642:errorcluster)  [unwired: 2 in, 2 out]
        n499 = local write "USB6218 Status"(w1634) -> ()
        n500 = Unbundle By Name(w1635) -> ("ReadLeakDet?"=w1639:bool, "Labels"=w1633:string[])
        n501 = Array Size(array=w1633) -> (size(s)=w1638:i32)
        n502 = case shown="True" w1639 {
          tunnel: w1638 -> [w1645 w1647]
          tunnel: [w1645 w1646] -> w1636
          frame False {
          }
          frame True {
            n503 = Add(x=w1647, y=1) -> (x+y=w1646:i32)
          }
        }
        n504 = Initialize Array(TRUE ("Activate 2"), w1636) -> ()  [unwired: 1 out]
      }
    }
    "error out (USB6218)" <- w886
    n505 = case shown="True" w848 {
      frame False {
      }
      frame True {
        n506 = local read "RUN label"() -> (w1025:string)
        n507 = Get Date/Time In Seconds() -> (seconds since 1Jan1904=w1029:timestamp)
        n508 = call "LV_UNIXTIME.vi"("current time"=w1029) -> ("date/time string"=w1028:string)  [unwired: 9 in, 1 out]
        n509 = Concatenate Strings(w1028, "_" ("string"), w1025) -> (→"RUN Identifier" →"RUN Identifier 2" →"RUN Identifier 3" →"RUN Identifier 4" →"RUN Identifier 5" →"RUN Identifier 6" →"RUN Identifier 7":string)
      }
    }
    n510 = Equal?(x=w858, y=i64 0) -> (x = y?=w855:bool)
    n511 = local read "LastData (LSI218)"() -> (w868:dbl[])
    n512 = local read "Last Data \nLSI336"() -> (w867:dbl[])
    n513 = And(x="Analog Out ON?", y=w848) -> (x .and. y?=w884:bool)
    n514 = And(x=w855, y="Automatic \nScreenshots?") -> (x .and. y?=w854:bool)
    n515 = Build Array (concatenate)(w868, w867) -> (w866:dbl[])
    "AllTemperatures" <- w866
    n516 = Build Array (concatenate)(w870, w871) -> (w869:T18)
    "TempSensorsLocations" <- w869
    n517 = case shown="True" w884 {
      tunnel: w845 -> [_ w1418]
      tunnel: [w1394 w1409] -> w883
      tunnel: w882 -> [w1394 w1408]
      frame False {
      }
      frame True {
        w1401 = "_raw" ("string")
        w1425 = 10.0 ("V_lim_max")
        w1424 = 0.0 ("V_lim_min")
        w1423 = -1 items=["Default"=-1, "RSE"=10083, "Differential"=10106, "Pseudodifferential"=12529] ("output terminal configuration")
        w1422 = 10348 items=["Volts"=10348, "From Custom Scale"=10065] ("units")
        n518 = local read "RUN Identifier"() -> (w1407:string)
        n519 = Concatenate Strings(w1407, "_AO" ("string")) -> (w1427:string)
        n520 = Concatenate Strings(w1407, "_", "USB_AOUT.csv" ("string")) -> (w1419:string)
        n521 = Array To Cluster(array="AOUT Labels") -> (cluster=w1405:T28)
        n522 = Unbundle By Name(w1405) -> ("AOUT Labels[0]"=w1404:string, "AOUT Labels[1]"=w1402:string)
        n523 = Build Path(base path=w1418, name or relative path=w1419) -> (appended path=w1415:path)
        n524 = Concatenate Strings(w1404, w1401) -> (w1403:string)
        n525 = Concatenate Strings(w1402, w1401) -> (w1400:string)
        n526 = Open/Create/Replace File(file path (use dialog)=w1415, operation (0:open)=T24."open or create") -> (refnum out=w1413:refnum<file>)  [unwired: 4 in, 2 out]
        n527 = Build Array(w1404, w1402, w1403, w1400) -> (w1411:string[])
        n528 = call "FileIntialize.vi"("Error In"=w1408, "Labels"=w1411, "refnum in"=w1413) -> ("Error Out"=w1410:errorcluster, "File Refnum"=→"File Refn USB AO":refnum<file>)  [unwired: 7 in]
        n529 = call <vilib>:"DAQmx Create Task.vi"("new task name"=w1427, "auto cleanup"=FALSE, "error in"=w1410) -> ("task out"=w1426:refnum<k21>, "error out"=w1428:errorcluster)  [unwired: 11 in]
        n530 = Index Array(array="AOUT assignment", index #1=0 ("index"), index #2=1 ("index")) -> (element #1=w1397:tag, element #2=w1395:tag)
        n531 = call-poly <vilib>:"DAQmx Create Virtual Channel.vi"("task in"=w1426, "maximum value"=w1425, "minimum value"=w1424, "output terminal configuration"=w1423, "physical channels"=w1397, "units"=w1422, "error in"=w1428) -> ("task out"=w1430:refnum<k21>, "error out"=w1431:errorcluster)  [unwired: 7 in]
        n532 = call-poly <vilib>:"DAQmx Create Virtual Channel.vi"("task in"=w1430, "maximum value"=w1425, "minimum value"=w1424, "physical channels"=w1395, "error in"=w1431) -> ("task out"=w1433:refnum<k21>, "error out"=w1432:errorcluster)  [unwired: 9 in]
        n533 = call <vilib>:"DAQmx Start Task.vi"("task/channels in"=w1433, "error in"=w1432) -> ("task out"=→"AO task out":refnum<k21>, "error out"=w1409:errorcluster)  [unwired: 12 in]
      }
    }
    "error out (USB6210/6218 AOUT)" <- w883
    n534 = case shown="True" w854 {
      frame False {
      }
      frame True {
        n535 = flat-sequence {
          frame #0 {
            n536 = property on="Frontpanel screenshots" class="Bool (strict)"("Val(Sgnl)"=TRUE ("Value (Signaling)")) -> ()  [unwired: 2 in, 2 out]
          }
        }
      }
    }
    n537 = flat-sequence {
      tunnel: w866 -> [w1035]
      tunnel: w869 -> [w1036]
      tunnel: w861 -> [w1288]
      tunnel: w860 -> [w1287]
      frame #0 {
        n538 = stacked-sequence {
          tunnel: w1036 -> [w1041 w1046 w1051 w1056 w1061 w1066 w1071 w1076 w1081 w1086 w1091 w1096 w1101 w1106 w1111 w1116 w1121 w1126 w1131 w1136 w1141 w1146 w1151 w1156 w1161 w1166 w1171 w1176 w1181 w1186 w1191 w1196 w1201 w1206 w1211 w1216 w1221 w1226 w1231 w1236 w1241 w1246 w1251 w1256 w1261 w1266 w1271 w1276 w1281 w1286]
          tunnel: w1035 -> [w1039 w1044 w1049 w1054 w1059 w1064 w1069 w1074 w1079 w1084 w1089 w1094 w1099 w1104 w1109 w1114 w1119 w1124 w1129 w1134 w1139 w1144 w1149 w1154 w1159 w1164 w1169 w1174 w1179 w1184 w1189 w1194 w1199 w1204 w1209 w1214 w1219 w1224 w1229 w1234 w1239 w1244 w1249 w1254 w1259 w1264 w1269 w1274 w1279 w1284]
          frame #0 {
            n539 = Search 1D Array(1D array=w1041, element=T14."T3He1-1" ("SensorLocations")) -> (index of element=w1038:i32)  [unwired: 1 in]
            n540 = Index Array(array=w1039, index=w1038) -> (element=→"T3He1-1":dbl)
          }
          frame #1 {
            n541 = Search 1D Array(1D array=w1046, element=T14."T3He1-2" ("SensorLocations")) -> (index of element=w1043:i32)  [unwired: 1 in]
            n542 = Index Array(array=w1044, index=w1043) -> (element=→"T3He1-2":dbl)
          }
          frame #2 {
            n543 = Search 1D Array(1D array=w1051, element=T14."T3He1-3" ("SensorLocations")) -> (index of element=w1048:i32)  [unwired: 1 in]
            n544 = Index Array(array=w1049, index=w1048) -> (element=→"T3He1-3":dbl)
          }
          frame #3 {
            n545 = Search 1D Array(1D array=w1056, element=T14."T3He1-4" ("SensorLocations")) -> (index of element=w1053:i32)  [unwired: 1 in]
            n546 = Index Array(array=w1054, index=w1053) -> (element=→"T3He1-4":dbl)
          }
          frame #4 {
            n547 = Search 1D Array(1D array=w1061, element=T14."T3He2-1" ("SensorLocations")) -> (index of element=w1058:i32)  [unwired: 1 in]
            n548 = Index Array(array=w1059, index=w1058) -> (element=→"T3He2-1":dbl)
          }
          frame #5 {
            n549 = Search 1D Array(1D array=w1066, element=T14."T3He2-2" ("SensorLocations")) -> (index of element=w1063:i32)  [unwired: 1 in]
            n550 = Index Array(array=w1064, index=w1063) -> (element=→"T3He2-2":dbl)
          }
          frame #6 {
            n551 = Search 1D Array(1D array=w1071, element=T14."T3He3" ("SensorLocations")) -> (index of element=w1068:i32)  [unwired: 1 in]
            n552 = Index Array(array=w1069, index=w1068) -> (element=→"T3He3":dbl)
          }
          frame #7 {
            n553 = Search 1D Array(1D array=w1076, element=T14."T3He4" ("SensorLocations")) -> (index of element=w1073:i32)  [unwired: 1 in]
            n554 = Index Array(array=w1074, index=w1073) -> (element=→"T3He4":dbl)
          }
          frame #8 {
            n555 = Search 1D Array(1D array=w1081, element=T14."T3He5" ("SensorLocations")) -> (index of element=w1078:i32)  [unwired: 1 in]
            n556 = Index Array(array=w1079, index=w1078) -> (element=→"T3He5":dbl)
          }
          frame #9 {
            n557 = Search 1D Array(1D array=w1086, element=T14."T3He6-1" ("SensorLocations")) -> (index of element=w1083:i32)  [unwired: 1 in]
            n558 = Index Array(array=w1084, index=w1083) -> (element=→"T3He6-1" →"T3He6-1/6-2 (HEX1)":dbl)
          }
          frame #10 {
            n559 = Search 1D Array(1D array=w1091, element=T14."T3He6-2" ("SensorLocations")) -> (index of element=w1088:i32)  [unwired: 1 in]
            n560 = Index Array(array=w1089, index=w1088) -> (element=→"T3He6-2" →"T3He6-1/6-2 (3He pot) 2":dbl)
          }
          frame #11 {
            n561 = Search 1D Array(1D array=w1096, element=T14."T3He7-1" ("SensorLocations")) -> (index of element=w1093:i32)  [unwired: 1 in]
            n562 = Index Array(array=w1094, index=w1093) -> (element=→"T3He7-1" →"T3He7-1/7-2 (HEX1)":dbl)
          }
          frame #12 {
            n563 = Search 1D Array(1D array=w1101, element=T14."T3He7-2" ("SensorLocations")) -> (index of element=w1098:i32)  [unwired: 1 in]
            n564 = Index Array(array=w1099, index=w1098) -> (element=→"T3He7-2" →"T3He7-1/6-2 (3He pot) 2":dbl)
          }
          frame #13 {
            n565 = Search 1D Array(1D array=w1106, element=T14."T3He8" ("SensorLocations")) -> (index of element=w1103:i32)  [unwired: 1 in]
            n566 = Index Array(array=w1104, index=w1103) -> (element=→"T3He8":dbl)
          }
          frame #14 {
            n567 = Search 1D Array(1D array=w1111, element=T14."T3He9" ("SensorLocations")) -> (index of element=w1108:i32)  [unwired: 1 in]
            n568 = Index Array(array=w1109, index=w1108) -> (element=→"T3He9":dbl)
          }
          frame #15 {
            n569 = Search 1D Array(1D array=w1116, element=T14."T3He10" ("SensorLocations")) -> (index of element=w1113:i32)  [unwired: 1 in]
            n570 = Index Array(array=w1114, index=w1113) -> (element=→"T3He10":dbl)
          }
          frame #16 {
            n571 = Search 1D Array(1D array=w1121, element=T14."T4He1" ("SensorLocations")) -> (index of element=w1118:i32)  [unwired: 1 in]
            n572 = Index Array(array=w1119, index=w1118) -> (element=→"T4He1" →"T4He1 (4K reservoir )":dbl)
          }
          frame #17 {
            n573 = Search 1D Array(1D array=w1126, element=T14."T4He2-1" ("SensorLocations")) -> (index of element=w1123:i32)  [unwired: 1 in]
            n574 = Index Array(array=w1124, index=w1123) -> (element=→"T4He2-1":dbl)
          }
          frame #18 {
            n575 = Search 1D Array(1D array=w1131, element=T14."T4He2-2" ("SensorLocations")) -> (index of element=w1128:i32)  [unwired: 1 in]
            n576 = Index Array(array=w1129, index=w1128) -> (element=→"T4He2-2":dbl)
          }
          frame #19 {
            n577 = Search 1D Array(1D array=w1136, element=T14."T4He3-1" ("SensorLocations")) -> (index of element=w1133:i32)  [unwired: 1 in]
            n578 = Index Array(array=w1134, index=w1133) -> (element=→"T4He3-1":dbl)
          }
          frame #20 {
            n579 = Search 1D Array(1D array=w1141, element=T14."T4He3-2" ("SensorLocations")) -> (index of element=w1138:i32)  [unwired: 1 in]
            n580 = Index Array(array=w1139, index=w1138) -> (element=→"T4He3-2":dbl)
          }
          frame #21 {
            n581 = Search 1D Array(1D array=w1146, element=T14."T4He3-3" ("SensorLocations")) -> (index of element=w1143:i32)  [unwired: 1 in]
            n582 = Index Array(array=w1144, index=w1143) -> (element=→"T4He3-3":dbl)
          }
          frame #22 {
            n583 = Search 1D Array(1D array=w1151, element=T14."T4He3-4" ("SensorLocations")) -> (index of element=w1148:i32)  [unwired: 1 in]
            n584 = Index Array(array=w1149, index=w1148) -> (element=→"T4He3-4":dbl)
          }
          frame #23 {
            n585 = Search 1D Array(1D array=w1156, element=T14."T4He4" ("SensorLocations")) -> (index of element=w1153:i32)  [unwired: 1 in]
            n586 = Index Array(array=w1154, index=w1153) -> (element=→"T4He4":dbl)
          }
          frame #24 {
            n587 = Search 1D Array(1D array=w1161, element=T14."T4He5" ("SensorLocations")) -> (index of element=w1158:i32)  [unwired: 1 in]
            n588 = Index Array(array=w1159, index=w1158) -> (element=→"T4He5":dbl)
          }
          frame #25 {
            n589 = Search 1D Array(1D array=w1166, element=T14."T4He6" ("SensorLocations")) -> (index of element=w1163:i32)  [unwired: 1 in]
            n590 = Index Array(array=w1164, index=w1163) -> (element=→"T4He6":dbl)
          }
          frame #26 {
            n591 = Search 1D Array(1D array=w1171, element=T14."T4He7" ("SensorLocations")) -> (index of element=w1168:i32)  [unwired: 1 in]
            n592 = Index Array(array=w1169, index=w1168) -> (element=→"T4He7":dbl)
          }
          frame #27 {
            n593 = Search 1D Array(1D array=w1176, element=T14."T4He8" ("SensorLocations")) -> (index of element=w1173:i32)  [unwired: 1 in]
            n594 = Index Array(array=w1174, index=w1173) -> (element=→"T4He8":dbl)
          }
          frame #28 {
            n595 = Search 1D Array(1D array=w1181, element=T14."T4He9" ("SensorLocations")) -> (index of element=w1178:i32)  [unwired: 1 in]
            n596 = Index Array(array=w1179, index=w1178) -> (element=→"T4He9":dbl)
          }
          frame #29 {
            n597 = Search 1D Array(1D array=w1186, element=T14."T4He10" ("SensorLocations")) -> (index of element=w1183:i32)  [unwired: 1 in]
            n598 = Index Array(array=w1184, index=w1183) -> (element=→"T4He10":dbl)
          }
          frame #30 {
            n599 = Search 1D Array(1D array=w1191, element=T14."T1K1" ("SensorLocations")) -> (index of element=w1188:i32)  [unwired: 1 in]
            n600 = Index Array(array=w1189, index=w1188) -> (element=→"T1K1":dbl)
          }
          frame #31 {
            n601 = Search 1D Array(1D array=w1196, element=T14."T1K2" ("SensorLocations")) -> (index of element=w1193:i32)  [unwired: 1 in]
            n602 = Index Array(array=w1194, index=w1193) -> (element=→"T1K2":dbl)
          }
          frame #32 {
            n603 = Search 1D Array(1D array=w1201, element=T14."T1K3-1" ("SensorLocations")) -> (index of element=w1198:i32)  [unwired: 1 in]
            n604 = Index Array(array=w1199, index=w1198) -> (element=→"T1K3-1" →"T1K3-1/3-2 (1K pot)":dbl)
          }
          frame #33 {
            n605 = Search 1D Array(1D array=w1206, element=T14."T1K3-2" ("SensorLocations")) -> (index of element=w1203:i32)  [unwired: 1 in]
            n606 = Index Array(array=w1204, index=w1203) -> (element=→"T1K3-2" →"T1K3-1/3-2 (1K pot) 2":dbl)
          }
          frame #34 {
            n607 = Search 1D Array(1D array=w1211, element=T14."T1K4" ("SensorLocations")) -> (index of element=w1208:i32)  [unwired: 1 in]
            n608 = Index Array(array=w1209, index=w1208) -> (element=→"T1K4":dbl)
          }
          frame #35 {
            n609 = Search 1D Array(1D array=w1216, element=T14."T1K5" ("SensorLocations")) -> (index of element=w1213:i32)  [unwired: 1 in]
            n610 = Index Array(array=w1214, index=w1213) -> (element=→"T1K5":dbl)
          }
          frame #36 {
            n611 = Search 1D Array(1D array=w1221, element=T14."T1K6" ("SensorLocations")) -> (index of element=w1218:i32)  [unwired: 1 in]
            n612 = Index Array(array=w1219, index=w1218) -> (element=→"T1K6":dbl)
          }
          frame #37 {
            n613 = Search 1D Array(1D array=w1226, element=T14."TIP1" ("SensorLocations")) -> (index of element=w1223:i32)  [unwired: 1 in]
            n614 = Index Array(array=w1224, index=w1223) -> (element=→"TIP1":dbl)
          }
          frame #38 {
            n615 = Search 1D Array(1D array=w1231, element=T14."TIP2" ("SensorLocations")) -> (index of element=w1228:i32)  [unwired: 1 in]
            n616 = Index Array(array=w1229, index=w1228) -> (element=→"TIP2":dbl)
          }
          frame #39 {
            n617 = Search 1D Array(1D array=w1236, element=T14."TIP3" ("SensorLocations")) -> (index of element=w1233:i32)  [unwired: 1 in]
            n618 = Index Array(array=w1234, index=w1233) -> (element=→"TIP3":dbl)
          }
          frame #40 {
            n619 = Search 1D Array(1D array=w1241, element=T14."TIP4" ("SensorLocations")) -> (index of element=w1238:i32)  [unwired: 1 in]
            n620 = Index Array(array=w1239, index=w1238) -> (element=→"TIP4":dbl)
          }
          frame #41 {
            n621 = Search 1D Array(1D array=w1246, element=T14."TIP5" ("SensorLocations")) -> (index of element=w1243:i32)  [unwired: 1 in]
            n622 = Index Array(array=w1244, index=w1243) -> (element=→"TIP5":dbl)
          }
          frame #42 {
            n623 = Search 1D Array(1D array=w1251, element=T14."TIP6" ("SensorLocations")) -> (index of element=w1248:i32)  [unwired: 1 in]
            n624 = Index Array(array=w1249, index=w1248) -> (element=→"TIP6":dbl)
          }
          frame #43 {
            n625 = Search 1D Array(1D array=w1256, element=T14."TIP7" ("SensorLocations")) -> (index of element=w1253:i32)  [unwired: 1 in]